vi "OFDM_Rx_5.0.vi"() -> ()   [LabVIEW 2015]
uses:
  <vilib>/imath/engines/lvmath/Plug In/_Char/NIMS_CH_character datatype.ctl
  <vilib>/Analysis/2dsp.llb/Complex FFT.vi
  <instrlib>/niUSRP/niUSRP Fetch Rx Data (CDB Cluster).vi
  <vilib>/imath/engines/lvmath2/RunTimeEngine/BuiltInFunctions/figure/NIMS_figure.vi
  <vilib>/imathl/engines/lvmath/Functions/Error Handling/Create Error.vi
  <vilib>/imath/engines/lvmath2/RunTimeEngine/IndexRead/NIMS V(S).vi
  <instcachedir>/0/NIMS V(S)_0488751826AF41519A22953C041130DC.lvgen/NIMS V(S)_0488751826AF41519A22953C041130DC_002.vi
  <vilib>/imath/engines/lvmath2/RunTimeEngine/IndexRead/NIMS V(R2).vi
  <instcachedir>/0/NIMS V(R2)_C76619605A0E4E9F8B2FA9389712AC47.lvgen/NIMS V(R2)_C76619605A0E4E9F8B2FA9389712AC47_001.vi
  <vilib>/imath/engines/lvmath2/RunTimeEngine/BuiltInFunctions/abs/NIMS_abs(signed).vi
  <instcachedir>/0/NIMS_abs(signed)_C4FCB8E6058B49B797C7C8D53CA5F6EC.lvgen/NIMS_abs(signed)_C4FCB8E6058B49B797C7C8D53CA5F6EC_006.vi
  <vilib>/imath/engines/lvmath2/RunTimeEngine/ErrorHandling/NIMS_Create Error From Enums.vi
  <vilib>/imath/engines/lvmath2/RunTimeEngine/BuiltInFunctions/plot/NIMS_plot(G, Str).vi
  <instcachedir>/0/NIMS_plot(G, Str)_4C4ED324FCF14F2FB79D7E74DE209E0D.lvgen/NIMS_plot(G, Str)_4C4ED324FCF14F2FB79D7E74DE209E0D_000.vi
  <vilib>/imath/engines/lvmath/Plug In/_Char/NIMS_CH_Character RV to String.vi
  <vilib>/imath/engines/lvmath2/RunTimeEngine/BuiltInFunctions/title/NIMS_title.vi
  <vilib>/imath/engines/lvmath2/RunTimeEngine/BuiltInFunctions/xlabel/NIMS_xlabel.vi
  <vilib>/imath/engines/lvmath2/RunTimeEngine/BuiltInFunctions/ylabel/NIMS_ylabel.vi
  <vilib>/imath/engines/lvmath2/RunTimeEngine/BuiltInFunctions/view_image/NIMS_view_image.vi
  <vilib>/imath/engines/lvmath2/RunTimeEngine/ErrorHandling/NIMS_Finalize Error.vi
  <vilib>/Analysis/NI_AALPro.lvlib
panel:
  in  "Symbol Rate (sym/sec)":i16=10000
  out "coerced gain":dbl format="%#_6f"
  out "coerced carrier frequency":dbl=2422000000.004802 format="%#_6p"
  out "coerced IQ rate":dbl=7692307.692307692 format="%#_6p"
  out "error out":errorcluster
  in  "IQ rate":dbl=8000000.0 format="%#_6p"
  in  "Gain (dB)":dbl format="%#_6f"
  in  "RX antenna":string="RX2"
  in  "Carrier Frequency (Hz)":dbl=2422000000.0 format="%#_6p"
  in  "RX Device":refnum<k15>="192.168.10.2"
  in  "cp_length":i16=28
  in  "frame_length":i64=220
  in  "pilot_offset_time":i16=4
  in  "pilot_offset_freq":i16=12
  in  "pilot_start":i16=2
  in  "SC_pilot":i16=18
  in  "SC_data":i64=180
  in  "SC_total":i16=256
  out "recvd":cdb[](array[numeric])
  out "Demod Bits":i8[](array[numeric])
  out "H_est":cdb[](array[numeric])=[0.08958843473744027+0.033866919628362226i, 0.08933306772511067+0.033754535815650154i, 0.0890796995797373+0.033689691127898796i, 0.088824457649056+0.033653137127223176i, 0.08856200140099749+0.03360892848502687i, 0.08828699030349248+0.03352111987271347i, 0.08799799560338455+0.03336623048653605i, 0.08770923566316845+0.03317063762214553i, 0.08743884062425179+0.03297318310004233i, 0.08720494062804221+0.03281270874072685i, 0.08701428721717738+0.032713813875976924i, 0.08682811753921568+0.03264412788268006i, 0.08659629014294555+0.03255703764900121i, 0.08626866357715542+0.032405930063105305i, 0.08581473246366589+0.032157612896037795i, 0.085282535716426+0.031832577450366245i, 0.08473974832241693+0.03146473591153873i, 0.08425404526861986+0.031088000465003315i, 0.08387212634944503+0.030735939318786848i, 0.08355679058901888+0.030440744771231237i, 0.08324986181889696+0.030234265143257145i, 0.08289316387063478+0.030148348755785252i, 0.08243918686965175+0.030190622708217187i, 0.08188308611682285+0.03027182921387839i, 0.08123068320688688+0.03027848926457527i, 0.08048779973458267+0.030097123852114233i, 0.07966894464577944+0.029651104883325022i, 0.07882337629086764+0.029011207925130747i, 0.07800904037136812+0.028285059459477867i, 0.07728388258880174+0.02758028596831284i, 0.07668786809215022+0.02698606150786384i, 0.07618903982023899+0.026517750431485982i, 0.07573746015935434+0.02617226466681609i, 0.07528319149578261+0.025946516141490985i, 0.0747807344237453+0.025827063555393253i, 0.07420234236920467+0.02575905269738841i, 0.07352470696605823+0.025677276128587716i, 0.0727245198482034+0.025516526410102446i, 0.07179448933316374+0.025227593777126724i, 0.07079139047296706+0.024825259161186136i, 0.06978801500326731+0.02434030116788915i, 0.06885715465971835+0.023803498402844212i, 0.06805393879867762+0.023247858329851913i, 0.06736284725931643+0.02271530384548135i, 0.06675069750150965+0.022249986704493758i, 0.06618430698513207+0.021896058661650366i, 0.06562627388725574+0.02167743556932108i, 0.06502231925374133+0.021537089670310573i, 0.06431394484764673+0.021397757305032176i, 0.0634426524320298+0.02118217481389923i, 0.062382234707500366+0.020832530912627954i, 0.061235648124876+0.020368823818146045i, 0.060138140072526276+0.019830504122684087i, 0.05922495793882071+0.019257022418472648i, 0.058583607324806844+0.01868700128024326i, 0.05811062668224429+0.018155751212731306i, 0.057654812675570634+0.017697754703173113i, 0.057064961969223484+0.017347494238805012i, 0.05623020375790453+0.017121044911569915i, 0.05520099735737172+0.016960852232237034i, 0.054068134613647116+0.016790954316282164i, 0.05292240737275276+0.0165353892791811i, 0.051844899309820516+0.016140824198598525i, 0.050877861416421644+0.01564444200095474i, 0.05005383651323721+0.015106054574858935i, 0.04940536742094827+0.014585473808920302i, 0.04894182541927298+0.014133720392977563i, 0.04857989562407772+0.013766650221787528i, 0.048213091610265935+0.013491327991336543i, 0.04773492695274108+0.013314818397610948i, 0.04706616326888732+0.01323266978241776i, 0.04623655434601177+0.013194365070846713i, 0.04530310201390224+0.013137870833808227i, 0.04432280810234655+0.013001153642212706i, 0.04335225277279916+0.012741541542414704i, 0.04244632951338097+0.012393808482545291i, 0.04165951014387954+0.01201208988617968i, 0.04104626648408239+0.011650521176893075i, 0.04063246262024927+0.011351566988290148i, 0.04032953170452874+0.011111008794093415i, 0.04002029915554156+0.010912957278054854i, 0.039587590391908484+0.010741523123926447i, 0.03894671055462557+0.010581861497317558i, 0.03814288367419006+0.010423305491267104i, 0.037253813503474495+0.01025623268067139i, 0.036357203795351414+0.010071020640426715i, 0.03552324102366187+0.00986346525558041i, 0.03479204254612094+0.009651035651783877i, 0.03419620844141226+0.009456619264839547i, 0.03376833878821942+0.009303103530549849i, 0.033518180035157344+0.009205483671154556i, 0.03336406411056614+0.009147186054642834i, 0.033201469312717245+0.00910374483544119i, 0.032925873939882076+0.00905069416797614i, 0.03246087176971073+0.008968878275898547i, 0.03184251849736791+0.008860381659756715i, 0.03113498529739702+0.008732598889323298i, 0.030402443344341435+0.008592924534370959i, 0.02970567904379864+0.008450433796661163i, 0.029091939725582557+0.008320924405910639i, 0.0286050879505612+0.008221874723824924i, 0.028288986279602583+0.00817076311210956i, 0.028161478393172047+0.008178112455157264i, 0.028136332450124167+0.008226623728109478i, 0.028101297728910835+0.008292042428794826i, 0.02794412350798395+0.008350114055041933i, 0.02758395524816432+0.008381154914829148i, 0.02706552313974841+0.008383764556733748i, 0.026464953555401592+0.008361113339482735i, 0.025858372867789255+0.008316371621803114i, 0.02531427250217544+0.00825716813400861i, 0.024870604094218852+0.008208965092759847i, 0.024557684332176855+0.008201683086304173i, 0.02440582990430682+0.00826524270288893i, 0.024422814793560607+0.008416997976839551i, 0.02452624216166803+0.00862403672679379i, 0.024611172465053396+0.008840880217467496i, 0.024572666160141015+0.009022049713576504i, 0.024336751916882216+0.009132361175597627i, 0.023953331259336443+0.009177809347051527i, 0.023503273925090162+0.009174683667219836i, 0.023067449651729834+0.009139273575384186i, 0.02271506188866966+0.00909169305519065i, 0.022468648932634776+0.009067354267743062i, 0.022339082792178055+0.009105493918509698i, 0.02233723547585236+0.009245348712958837i, 0.022459616561076624+0.009507764618171296i, 0.022645285900733995+0.009840024647678063i, 0.02281894091657368+0.010171021076622669i, 0.0229052790303449+0.010429646180148643i, 0.022849273298632313+0.010563397518747127i, 0.02267699931736241+0.010594193794299694i, 0.02243480831729715+0.010562558994035529i, 0.02216905152919847+0.010509017105183817i, 0.021925125223911116+0.010473135918277353i, 0.02174460583261099+0.010490658437063385i, 0.0216681148265568+0.010596371468592762i, 0.021736273677007242+0.010825061819916342i, 0.021968070506904646+0.011191479519267156i, 0.022295960045925864+0.011630227479606934i, 0.022630763675431386+0.012055871835079586i, 0.022883302776781685+0.012382978719829019i, 0.022989186555202858+0.012549863714924146i, 0.022983175511383368+0.012589840189133915i, 0.02292481796987731+0.012559970958152283i, 0.022873662255238757+0.012517318837673205i, 0.022880774882413423+0.012513897983773378i, 0.022963295127913567+0.012581527914060465i, 0.02312988045864309+0.012746979486524871i, 0.02338918834150588+0.013037023559157002i, 0.023739965939476717+0.013459240333087008i, 0.024141319199813882+0.013944447382004023i, 0.024542443765846543+0.014404271622736924i, 0.02489253528090386+0.01475033997211459i, 0.025155062326584304+0.014919712697919488i, 0.025350585237563585+0.014951183471748439i, 0.025513937286786713+0.014908979316151845i, 0.02567995174719871+0.014857327253680113i, 0.02588027391402679+0.014855214937099723i, 0.02613379717162701+0.014940672540041427i, 0.026456226926637634+0.015146490866352058i, 0.026863268585696914+0.015505460719878442i, 0.027361085362622693+0.016026529911111757i, 0.027917671699951137+0.016623274277120573i, 0.02849147984739799+0.017185426661617813i, 0.029040962054678997+0.017602719908316404i, 0.029533521156327937+0.01779619556884619i, 0.02997236232615067+0.017812130026504745i, 0.03036964132277111+0.017728108372506567i, 0.030737513904813146+0.017621715698066153i, 0.031092706826119025+0.017563999399143014i, 0.03147023082140438+0.017599856090676724i, 0.03190966762060318+0.01776764469235187i, 0.032450598953649434+0.01810572412385303i, 0.033117467092251524+0.018627241434810576i, 0.03387415647521555+0.01924449619463802i, 0.03466941208312203+0.01984457610269467i, 0.03545197889655147+0.020314568858339817i, 0.0361793221032264+0.020571613935626697i, 0.036843787719437415+0.020653057907384247i, 0.0374464419686171+0.020626299121135356i, 0.03798835107419805+0.020558735924402903i, 0.03847967823781341+0.020515249461351494i, 0.038966974573898555+0.02055065206271268i, 0.03950588817508943+0.020717238855859736i, 0.04015206713402196+0.02106730496816594i, 0.04094405145025874+0.021621672223258902i, 0.04185194875106904+0.022275269229783585i, 0.04282875857064877+0.022891551292639287i, 0.04382748044319387+0.023333973716725312i, 0.044800795021846994+0.023509409017171495i, 0.045700107435537755+0.02349839855002986i, 0.046476503932142504+0.023424900881582944i, 0.047081070759537595+0.023412874578113314i, 0.04749589253501365+0.023559068525366263i, 0.04782704735351838+0.02385139288693803i, 0.04821161167941378+0.024250548145887584i, 0.04878666197706183+0.024717234785273896i, 0.04964554560096747+0.025212450908722445i, 0.050706693466207445+0.025698385102124667i, 0.05184480737800145+0.0261375235719385i, 0.052934589141569184+0.026492352524621884i, 0.053879056780077435+0.02673491598917671i, 0.05469449318848138+0.026875489284780677i, 0.05542549747968328+0.026933905553155436i, 0.0561166687665854+0.02692999793602264i, 0.05680708811826002+0.026890202908053037i, 0.05751376442845945+0.026867370275713814i, 0.05824818854710604+0.02692095317842123i, 0.059021851324122125+0.027110404755591566i, 0.05984194260187441+0.027475976483276775i, 0.060698448192507144+0.02798111318407151i, 0.06157705290060896+0.028570058017206107i, 0.062463441530768486+0.029187054141910893i, 0.0633457106712277+0.02978574746686676i, 0.06422160404484167+0.03035739489855646i, 0.06509127715811858+0.03090265609291318i, 0.06595488551756731+0.03142219070587055i, 0.06681258462969608+0.03191665839336173i, 0.06766453000101327+0.03238671881132004i, 0.06851087713802709+0.03283303161567867i, 0.06935178154724642+0.033256256462371216i, 0.07018739873517946+0.03365705300733085i, 0.0710178842083346+0.03403608090649089i, 0.07184339347322007+0.034393999815784566i, 0.07266408203634472+0.03473146939114541i, 0.07348010540421678+0.03504914928850662i, 0.07429161908334461+0.03534769916380154i, 0.07509877858023645+0.03562777867296338i, 0.07590173940140113+0.03589004747192566i, 0.07670065705334692+0.03613516521662159i, 0.07749568704258218+0.0363637915629845i, 0.07828698487561511+0.036576586166947644i, 0.07907470605895459+0.03677420868444449i, 0.07985900609910884+0.03695731877140827i, 0.08064004050258625+0.0371265760837723i, 0.08141796477589523+0.03728264027746993i, 0.082192934425544+0.03742617100843442i, 0.08296510495804144+0.03755782793259918i, 0.08373463187989572+0.03767827070589749i, 0.08450167069761526+0.03778815898426266i, 0.08526637691770828+0.037888152423627995i, 0.08602890604668362+0.03797891067992687i, 0.08678941359104951+0.03806109340909257i, 0.08754805505731435+0.03813536026705842i, 0.08830498595198633+0.03820237090975773i, 0.08906036178157432+0.03826278499312384i, 0.08981433805258654+0.03831726217309007i, 0.0905670702715314+0.038366462105589735i, 0.09131871394491708+0.03841104444655613i, 0.09206942457925246+0.03845166885192263i, 0.09281935768104575+0.038488994977622516i, 0.09356866875680535+0.03852368247958912i, 0.09431751331303947+0.038556391013755756i, 0.09506604685625697+0.03858778023605577i, 0.09581442489296604+0.03861850980242244i]
  out "BER":dbl=0.000791094
  # "USRP PARAMETERS"
  # "OFDM PARAMETERS"
  # "PILOT DISTRIBUTION PARAMETERS"
  # "INDICATORS"
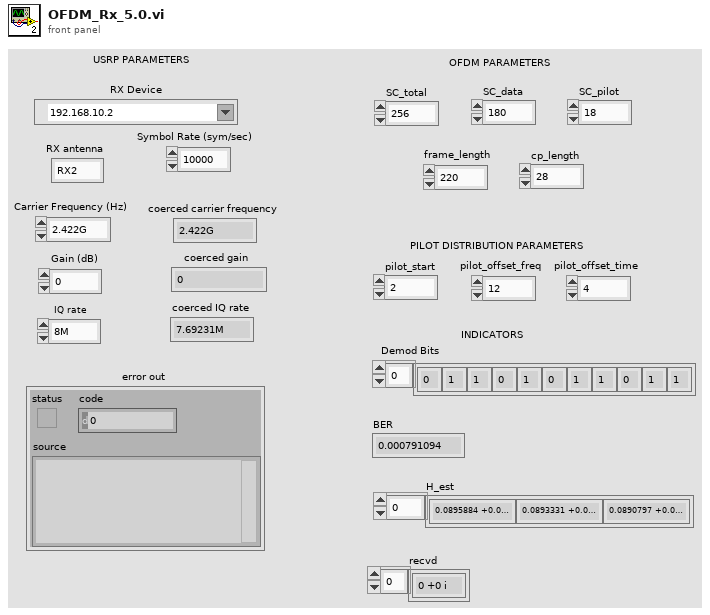
[diagram p1: front panel]
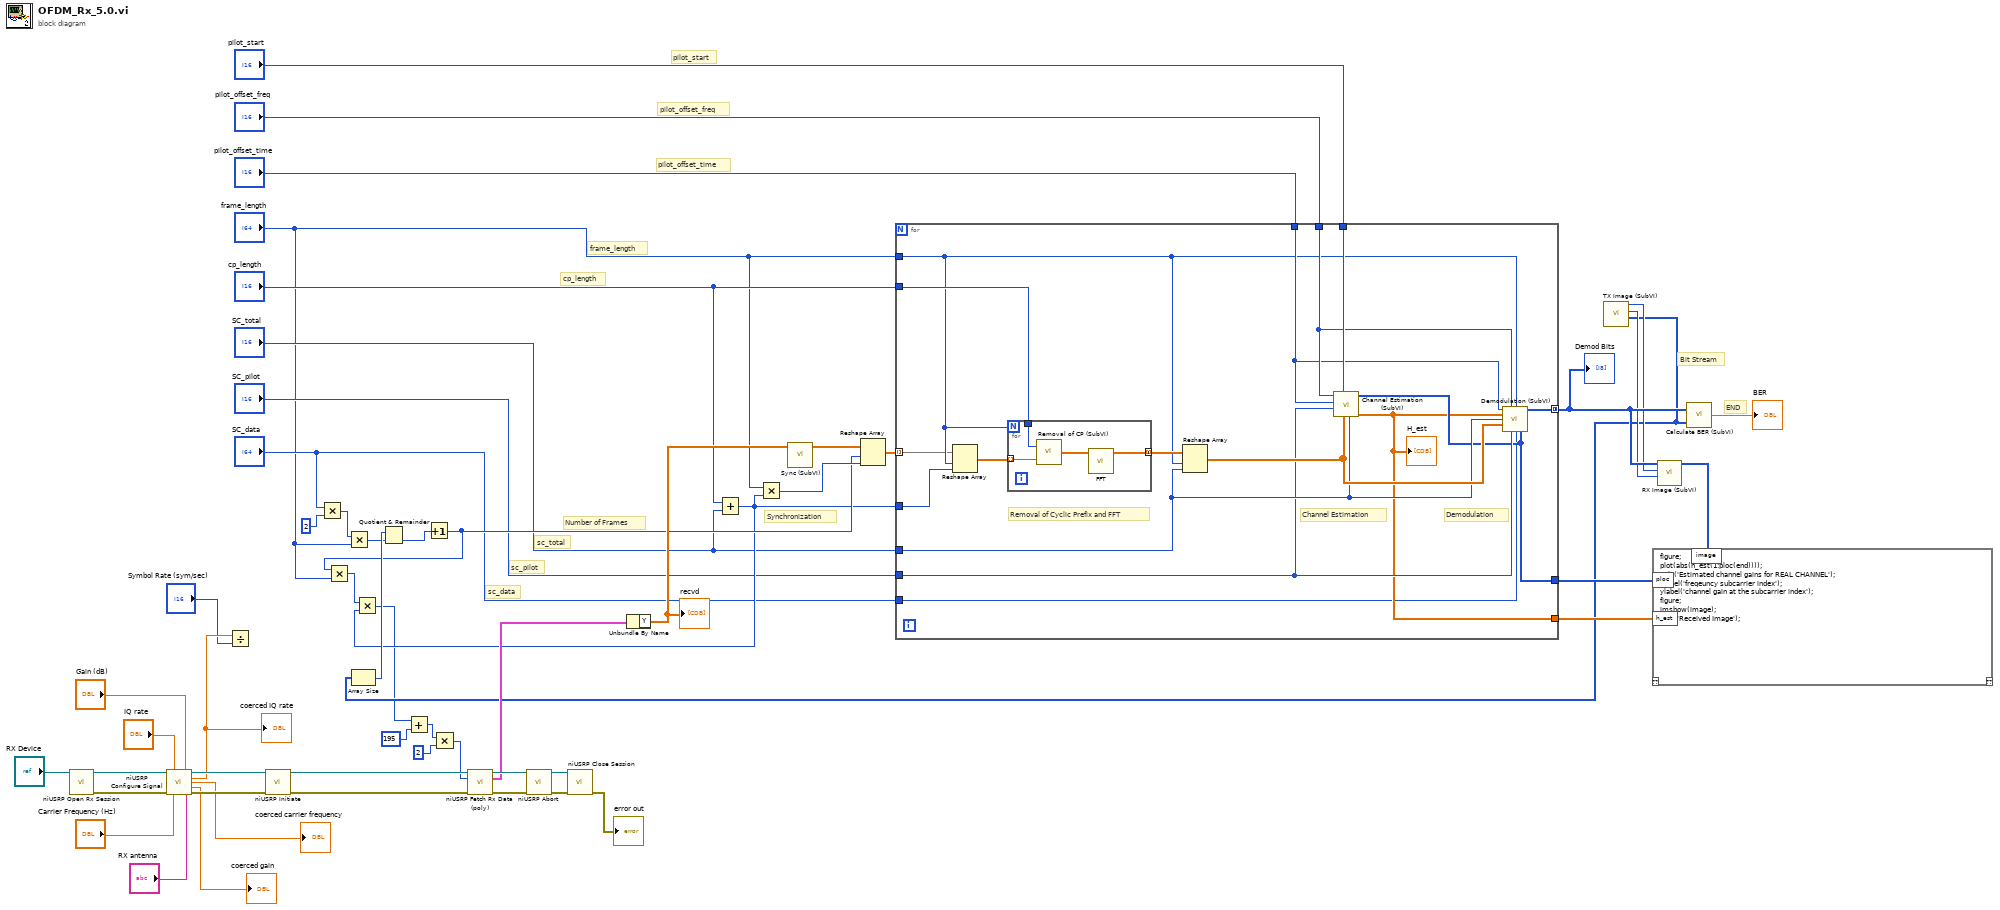
[diagram p0: block diagram]
diagram:
  # "Number of Frames"
  # "Synchronization"
  # "Bit Stream"
  # "pilot_offset_time"
  # "pilot_offset_freq"
  # "pilot_start"
  # "END"
  # "cp_length"
  # "frame_length"
  # "sc_total"
  # "sc_pilot"
  # "sc_data"
  n1 = call <instrlib>:"niUSRP Open Rx Session.vi"("device names"="RX Device") -> ("session handle out"=w46:refnum<k15>, "error out"=w45:errorcluster)  [unwired: 13 in]
  n2 = call <instrlib>:"niUSRP Configure Signal.vi"("session handle"=w46, "IQ rate"="IQ rate", "carrier frequency"="Carrier Frequency (Hz)", "gain"="Gain (dB)", "error in (no error)"=w45, "active antenna"="RX antenna") -> ("session handle out"=w44:refnum<k15>, "coerced IQ rate"=w7:dbl, "coerced carrier frequency"=→"coerced carrier frequency":dbl, "coerced gain"=→"coerced gain":dbl, "error out"=w43:errorcluster)  [unwired: 5 in]
  "coerced IQ rate" <- w7
  n3 = Divide(x=w7, y="Symbol Rate (sym/sec)") -> ()  [unwired: 1 out]
  n4 = call <instrlib>:"niUSRP Initiate.vi"("session handle"=w44, "error in (no error)"=w43) -> ("session handle out"=w40:refnum<k15>, "error out"=w37:errorcluster)  [unwired: 12 in]
  n5 = Multiply(x="SC_data", y=i64 2) -> (x*y=w26:i64)
  n6 = Multiply(x=w26, y="frame_length") -> (x*y=w27:i64)
  n7 = Add(x="cp_length", y="SC_total") -> (x+y=w20:i16)
  n8 = Multiply(x="frame_length", y=w20) -> (x*y=w51:i64)
  n9 = call "TX Image (SubVI).vi"() -> ("image_bits"=w25:i8[], "columns"=w31:i32, "rows"=w32:i32)  [unwired: 9 in]
  n10 = Array Size(array=w25) -> (size(s)=w29:i32)
  n11 = Quotient & Remainder(x=w29, y=w27) -> (floor(x/y)=w28:i64)  [unwired: 1 out]
  n12 = Increment(x=w28) -> (x+1=w22:i64)
  n13 = Multiply(x=w22, y="frame_length") -> (x*y=w21:i64)
  n14 = Multiply(x=w21, y=w20) -> (x*y=w19:i64)
  n15 = Add(x=w19, y=i64 195) -> (x+y=w23:i64)
  n16 = Multiply(x=w23, y=i64 2) -> (x*y=w34:i64)
  n17 = call-poly <instrlib>:"niUSRP Fetch Rx Data (poly).vi"("session handle"=w40, "number of samples"=w34, "error in (no error)"=w37) -> ("session handle out"=w39:refnum<k15>, "data"=w36:cluster{"t0":dbl, "dt":dbl, "Y":cdb[]}, "error out"=w38:errorcluster)  [unwired: 9 in, 1 out]
  n18 = call <instrlib>:"niUSRP Abort.vi"("session handle"=w39, "error in (no error)"=w38) -> ("session handle out"=w42:refnum<k15>, "error out"=w41:errorcluster)  [unwired: 12 in]
  n19 = call <instrlib>:"niUSRP Close Session.vi"("session handle"=w42, "error in (no error)"=w41) -> ("error out"=→"error out":errorcluster)  [unwired: 13 in]
  n20 = Unbundle By Name(w36) -> ("Y"=w33:cdb[])
  "recvd" <- w33
  n21 = call "Sync (SubVI).vi"("sampled\n   array"=w33) -> ("after_sync"=w47:cdb[])  [unwired: 10 in]
  n22 = Reshape Array(w47, w22, w51) -> (w50:cdb[][])
  n23 = for {
    tunnel: "cp_length" -> [w68]
    tunnel: "SC_total" -> [w67]
    tunnel: "pilot_start" -> [w66]
    tunnel: "pilot_offset_freq" -> [w65]
    tunnel: "pilot_offset_time" -> [w64]
    tunnel: [w62] -> w48 mode=concatenating
    tunnel: "SC_pilot" -> [w61]
    tunnel: [w60] -> w53
    tunnel: [w59] -> w52
    tunnel: "SC_data" -> [w58]
    tunnel: "frame_length" -> [w57]
    tunnel: w20 -> [w56]
    tunnel: w50 -> [w55] mode=indexing
    # "Demodulation"
    # "Channel Estimation"
    # "Removal of Cyclic Prefix and FFT"
    n24 = Reshape Array(w55, w57, w56) -> (w63:cdb[][])
    n25 = for {
      N: w57 -> [_]
      tunnel: w63 -> [w74] mode=indexing
      tunnel: w68 -> [w73]
      tunnel: [w71] -> w70 mode=concatenating
      n26 = call "Removal of CP (SubVI).vi"("ch_output in"=w74, "cp_length"=w73) -> ("ch_output out"=w72:cdb[])
      n27 = call-poly <vilib>:"FFT.vi"("X"=w72) -> ("FFT {X}"=w71:cdb[])  [unwired: 9 in, 1 out]
    }
    n28 = Reshape Array(w70, w57, w67) -> (w69:cdb[][])
    n29 = call "Channel Estimation (SubVI).vi"("SC_total"=w67, "ofdm_output"=w69, "pilot_start"=w66, "SC_pilot"=w61, "pilot_offset_time"=w64, "pilot_offset_freq"=w65) -> ("H_est"=w59:cdb[], "est_ploc_mtx"=w60:i32[])  [unwired: 1 in, 3 out]
    "H_est" <- w59
    n30 = call "Demodulation (SubVI).vi"("pilot_offset_time"=w64, "pilot_offset_freq"=w65, "frame_length"=w57, "H_est"=w59, "SC_total"=w67, "OFDM_output"=w69, "SC_pilot"=w61, "SC_data"=w58, "est_ploc_mtx"=w60) -> ("demod_data"=w62:i8[])  [unwired: 6 in]
  }
  "Demod Bits" <- w48
  n31 = call "RX Image (SubVI).vi"("columns"=w31, "rows"=w32, "Demod Bits"=w48) -> ("final_image"=w49:u8[][])  [unwired: 8 in]
  n32 = mathscript code="figure;\nplot(abs(h_est(1:ploc(end))));\ntitle('Estimated channel gains for REAL CHANNEL');\nxlabel('freqeuncy subcarrier index');\nylabel('channel gain at the subcarrier index');\nfigure;\nimshow(image);\ntitle('Received Image');"("h_est"=w52, "ploc"=w53, "image"=w49) -> ()  [unwired: 1 in, 1 out]
  n33 = call "Calculate BER (SubVI).vi"("Original Bits"=w25, "Demod Bits"=w48) -> ("BER"=→"BER":dbl)
